vi "Modelo planta H2_V2.vi"() -> ()   [LabVIEW 2024] (continued)
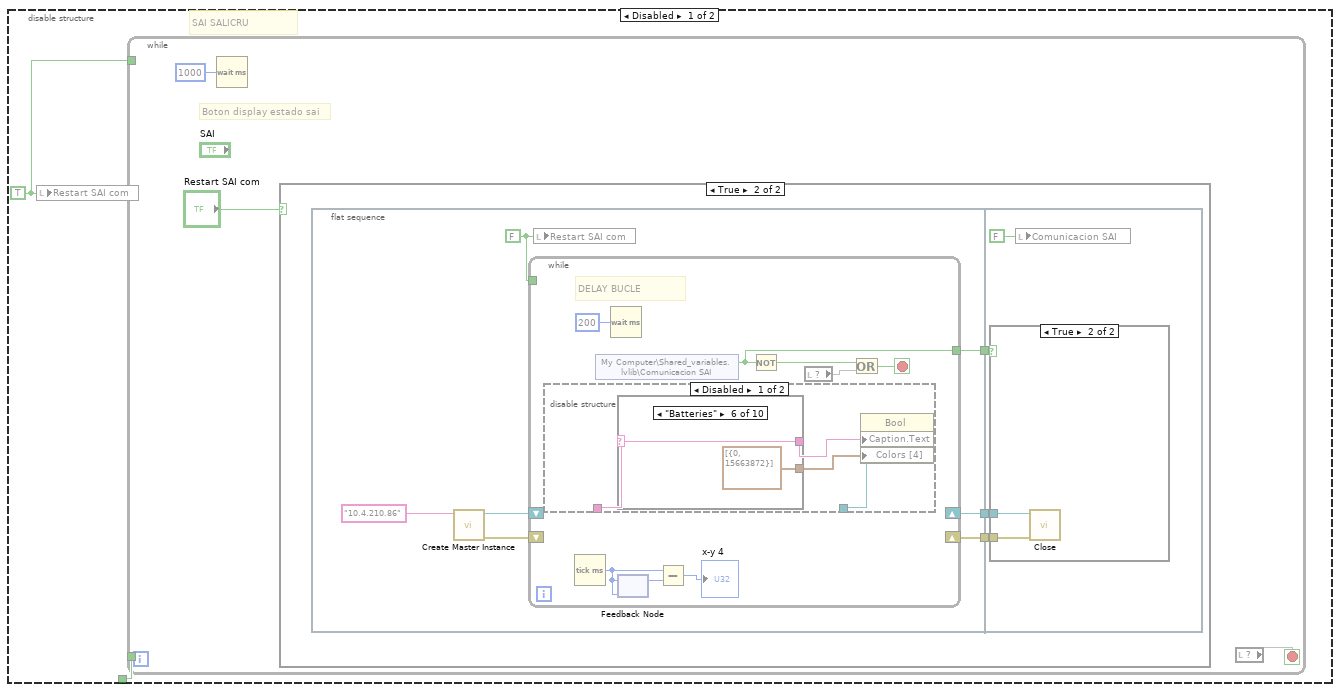
[diagram p2: hidden frame]
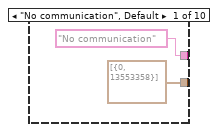
[diagram p4: hidden frame]
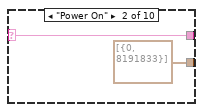
[diagram p5: hidden frame]
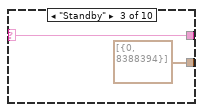
[diagram p6: hidden frame]
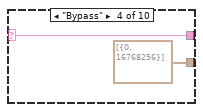
[diagram p7: hidden frame]
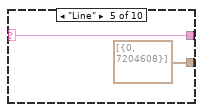
[diagram p8: hidden frame]
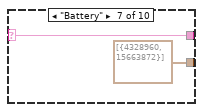
[diagram p9: hidden frame]
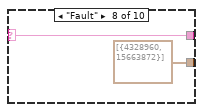
[diagram p10: hidden frame]
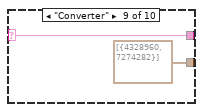
[diagram p11: hidden frame]
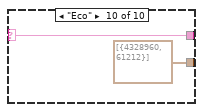
[diagram p12: hidden frame]
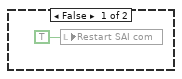
[diagram p14: hidden frame]
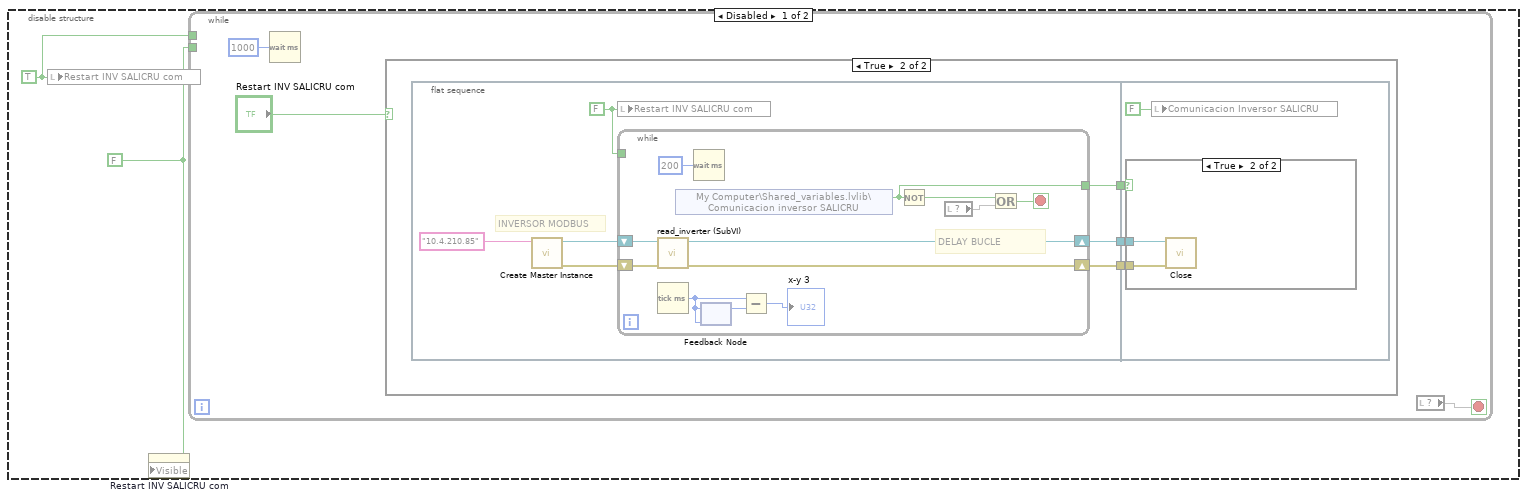
[diagram p15: hidden frame]
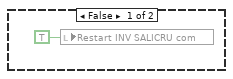
[diagram p17: hidden frame]
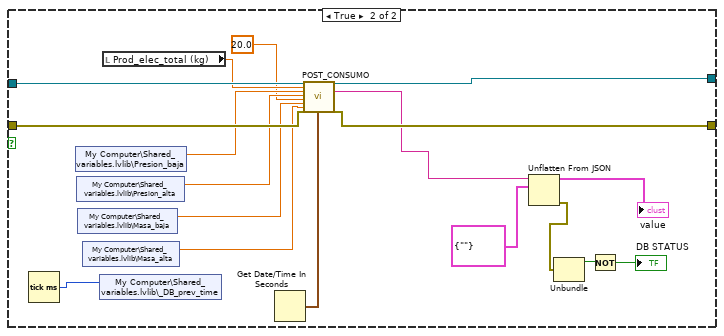
[diagram p18: hidden frame]
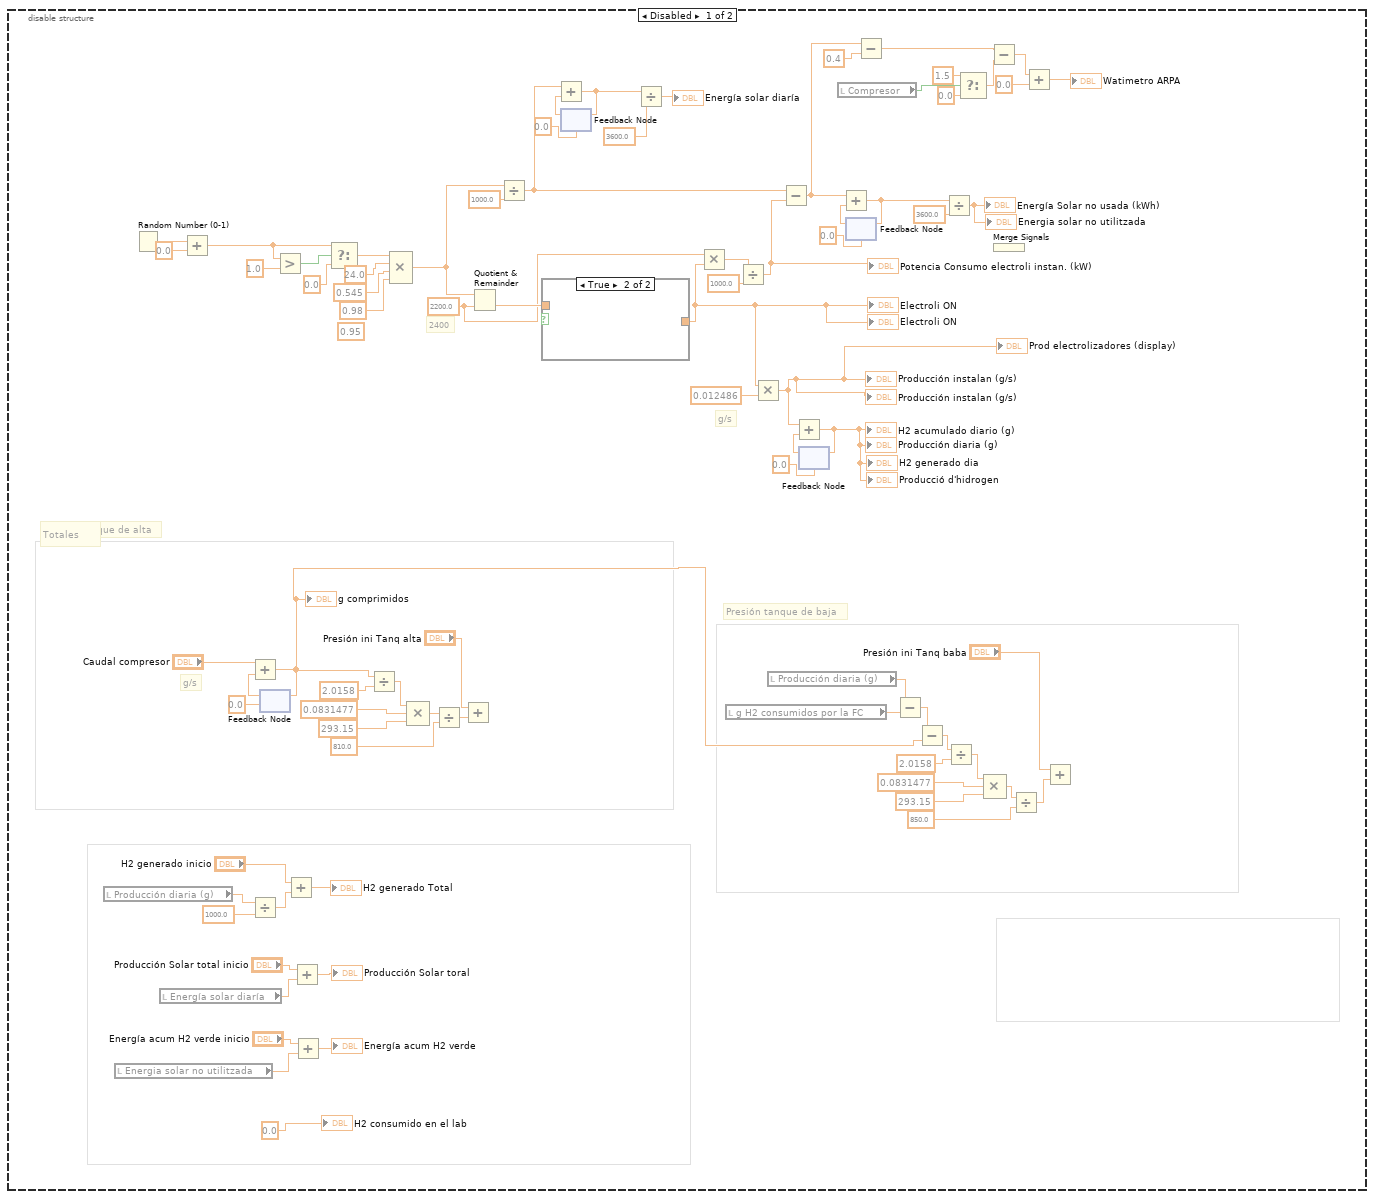
[diagram p20: hidden frame]
                    disable-tunnel: _ -> [w170 _]
                    disable-tunnel: _ -> [w167 _]
                    frame Disabled {
                      n87 = case shown="\"Batteries\"" w170 {
                        selector: w170 -> [_ w174 w176 w178 w180 w182 w184 w186 w188 w190]
                        tunnel: ["No communication" w174 w176 w178 w180 w182 w184 w186 w188 w190] -> w169
                        tunnel: [cluster{u32, u32}[] [{0, 13553358}] ("Colors [4]") cluster{u32, u32}[] [{0, 8191833}] ("Colors [4]") cluster{u32, u32}[] [{0, 8388394}] ("Colors [4]") cluster{u32, u32}[] [{0, 16768256}] ("Colors [4]") cluster{u32, u32}[] [{0, 7204608}] ("Colors [4]") cluster{u32, u32}[] [{0, 15663872}] ("Colors [4]") cluster{u32, u32}[] [{4328960, 15663872}] ("Colors [4]") cluster{u32, u32}[] [{4328960, 15663872}] ("Colors [4]") cluster{u32, u32}[] [{4328960, 7274282}] ("Colors [4]") cluster{u32, u32}[] [{4328960, 61212}] ("Colors [4]")] -> w168
                        frame "No communication", Default {
                        }
                        frame "Power On" {
                        }
                        frame "Standby" {
                        }
                        frame "Bypass" {
                        }
                        frame "Line" {
                        }
                        frame "Batteries" {
                        }
                        frame "Battery" {
                        }
                        frame "Fault" {
                        }
                        frame "Converter" {
                        }
                        frame "Eco" {
                        }
                      }
                      n88 = property class="Bool"(reference=w167, "Caption.Text"=w169, "Colors [4]"=w168) -> ()  [unwired: 1 in, 2 out]
                    }
                    frame Enabled {
                    }
                  }
                  n89 = Tick Count (ms)() -> (millisecond timer value=w164:u32)
                  n90 = shared-variable "My Computer\\Shared_variables.lvlib\\Comunicacion SAI"() -> (w160:bool)  [unwired: 1 in, 1 out]
                  n91 = Wait (ms)(milliseconds to wait=u32 200) -> ()  [unwired: 1 out]
                  n92 = feedback #6(w164) -> (w163:u32)
                  n93 = feedback-in #6(w164) -> ()
                  n94 = Subtract(x=w164, y=w163) -> (x-y=→"x-y 4":u32)
                  n95 = Not(x=w160) -> (.not. x?=w161:bool)
                  n96 = local read item#-1() -> (w159)
                  n97 = Or(x=w161, y=w159) -> (x .or. y?=w165:bool)
                }
                n98 = local write "Restart SAI com"(w153) -> ()
              }
              frame #1 {
                n99 = case shown="True" w191 {
                  tunnel: w194 -> [_ w197]
                  tunnel: w193 -> [_ w196]
                  frame False {
                    n100 = local write "Restart SAI com"(TRUE ("Restart SAI com")) -> ()
                  }
                  frame True {
                    n101 = call-dynamic "Close.vi"("error in (no error)"=w197, "Modbus master in"=w196) -> ()  [unwired: 9 in, 1 out]
                  }
                }
                n102 = local write "Comunicacion SAI"(FALSE) -> ()
              }
            }
          }
        }
        n103 = local read item#-1() -> (w146)
      }
    }
    frame Enabled {
    }
  }
  n104 = flat-sequence {
    tunnel: [w245] -> w26
    tunnel: [w240] -> w25
    tunnel: [w239] -> w24
    tunnel: [w220] -> w23
    tunnel: [map{string, dbl}[] []] -> w22
    tunnel: [w217] -> w21
    tunnel: [w216] -> w20
    tunnel: [w214] -> w19
    tunnel: [w213] -> w18
    tunnel: [w211] -> w17
    tunnel: [w210] -> w16
    tunnel: [w202] -> w15
    tunnel: [w201] -> w4
    tunnel: [w200] -> w3
    tunnel: w26 -> [_]
    tunnel: w25 -> [w269]
    tunnel: w24 -> [w270]
    tunnel: w23 -> [w252]
    tunnel: w22 -> [_]
    tunnel: w21 -> [w254]
    tunnel: w20 -> [w253]
    tunnel: w19 -> [w260]
    tunnel: w18 -> [w259]
    tunnel: w17 -> [w264]
    tunnel: w16 -> [w263]
    tunnel: w15 -> [w273]
    tunnel: [w268] -> w14
    tunnel: [w267] -> w13
    tunnel: [w266] -> w12
    tunnel: [w265] -> w11
    tunnel: [w261] -> w10
    tunnel: [w262] -> w9
    tunnel: [w258] -> w8
    tunnel: [w257] -> w7
    tunnel: [w256] -> w6
    tunnel: [w255] -> w5
    tunnel: w4 -> [w249]
    tunnel: w3 -> [w248]
    tunnel: [w247] -> w2
    tunnel: [w246] -> w1
    tunnel: w14 -> [w413]
    tunnel: w13 -> [w412]
    tunnel: w12 -> [w411]
    tunnel: w11 -> [w410]
    tunnel: w10 -> [w409]
    tunnel: w9 -> [w408]
    tunnel: w8 -> [w407]
    tunnel: w7 -> [w406]
    tunnel: w6 -> [w405]
    tunnel: w5 -> [w404]
    tunnel: w2 -> [w402]
    tunnel: w1 -> [w401]
    frame #0 {
      w244 = dynamicdata[] [] ("History Data")
      w245 = dbl[] [] ("History Data")
      # "INICIALIZACIÓN"
      n105 = property on="Restart SAI com" class="Bool (strict)"("Visible"=FALSE) -> ()  [unwired: 2 in, 2 out]
      n106 = Get Date/Time In Seconds() -> (seconds since 1Jan1904=w208:timestamp)
      n107 = control-ref of="E2.1"() -> (w230:refnum<vi>)
      n108 = control-ref of="E2.1.2"() -> (w231:refnum<vi>)
      n109 = control-ref of="E2.2"() -> (w233:refnum<vi>)
      n110 = control-ref of="E2.2.2"() -> (w234:refnum<vi>)
      n111 = control-ref of="E2.3.2"() -> (w236:refnum<vi>)
      n112 = control-ref of="E2.3"() -> (w237:refnum<vi>)
      n113 = control-ref of="E1.1,2"() -> (w226:refnum<vi>)
      n114 = control-ref of="E1.1"() -> (w225:refnum<vi>)
      n115 = control-ref of="E1.2"() -> (w223:refnum<vi>)
      n116 = control-ref of="E1.2.2"() -> (w222:refnum<vi>)
      n117 = control-ref of="E1.3.2"() -> (w227:refnum<vi>)
      n118 = control-ref of="E1.3"() -> (w228:refnum<vi>)
      n119 = Format Date/Time String(time format string (%c)="%Y_%m_%d_%H_%M", seconds (now)=w208) -> (date/time string=w206:string)  [unwired: 1 in]
      n120 = Build Array(w230, w231) -> (w232:refnum<vi>[])
      n121 = Build Array(w233, w234) -> (w235:refnum<vi>[])
      n122 = Build Array(w236, w237) -> (w238:refnum<vi>[])
      n123 = Build Array(w226, w225) -> (w224:refnum<vi>[])
      n124 = Build Array(w223, w222) -> (w221:refnum<vi>[])
      n125 = Build Array(w227, w228) -> (w229:refnum<vi>[])
      n126 = Build Array(w224, w221, w229, w232, w235, w238) -> (w220:refnum<vi>[][])
      n127 = Concatenate Strings("C:\\Users\\h2.lab\\Documents\\LabVIEW My DATA\\" ("string"), w206, "_data Planta Pilot.tdms" ("string")) -> (w207:string)
      n128 = call-poly <vilib>:"Create Master Instance.vi"("address"="10.4.210.79") -> ("error out"=w216:errorcluster, "TCP master instance"=w217:refnum<class "Modbus Master.lvclass">)  [unwired: 9 in]
      n129 = call-poly <vilib>:"Create Master Instance.vi"("address"="10.4.210.85") -> ("error out"=w213:errorcluster, "TCP master instance"=w214:refnum<class "Modbus Master.lvclass">)  [unwired: 9 in]
      n130 = call-poly <vilib>:"Create Master Instance.vi"("address"="10.4.210.86") -> ("error out"=w210:errorcluster, "TCP master instance"=w211:refnum<class "Modbus Master.lvclass">)  [unwired: 9 in]
      n131 = String To Path(string=w207) -> (path=w202:path)
      n132 = call <vilib>:"Connect.vi"("trust any server (F)"=TRUE, "security policy"=T2 {"message mode"=enum."None", "security"=enum."Basic256"}, "server endpoint URL"="opc.tcp://10.4.210.54:4841") -> ("error out"=w240:errorcluster, "OPC UA client refnum out"=w239:T7)  [unwired: 6 in, 1 out]
      n133 = property on="Potencia Solar Instanta (kW)" class="WFChart (strict)"("History Data"=w245) -> ()  [unwired: 2 in, 2 out]
      n134 = property on="Potencia Consumo electroli instan. (kW)" class="WFChart (strict)"("History Data"=w245) -> ()  [unwired: 2 in, 2 out]
      n135 = property on="Electroli ON" class="WFChart (strict)"("History Data"=w245) -> ()  [unwired: 2 in, 2 out]
      n136 = property on="Producción instalan (g/s)" class="WFChart (strict)"("History Data"=w245) -> ()  [unwired: 2 in, 2 out]
      n137 = property on="H2 acumulado diario (g)" class="WFChart (strict)"("History Data"=w245) -> ()  [unwired: 2 in, 2 out]
      n138 = property on="Energía Solar no usada (kWh)" class="WFChart (strict)"("History Data"=w245) -> ()  [unwired: 2 in, 2 out]
      n139 = property on="P tanq baja (barg)" class="WFChart (strict)"("History Data"=w245) -> ()  [unwired: 2 in, 2 out]
      n140 = property on="Producció d'hidrogen" class="WFChart (strict)"("History Data"=w245) -> ()  [unwired: 2 in, 2 out]
      n141 = property on="Energia solar no utilitzada" class="WFChart (strict)"("History Data"=w245) -> ()  [unwired: 2 in, 2 out]
      n142 = property on="Potència inversor solar" class="WFChart (strict)"("History Data"=w244) -> ()  [unwired: 2 in, 2 out]
      n143 = property on="Pressió tanc baixa" class="WFChart (strict)"("History Data"=w244) -> ()  [unwired: 2 in, 2 out]
      n144 = call "Init.vi"("Port"=u32 8000, "IP"="10.4.210.42") -> ("error out"=w200:errorcluster, "DB_API.lvclass 2"=w201:refnum<class "DB_API.lvclass">)  [unwired: 8 in]
    }
    frame #1 {
      # "PLC"
      # "ELECTROLIZADORES"
      # "ALMACENAMIENTO DE DATOS"
      n145 = node-c288() -> (w275:T3)  [unwired: 4 in]
      n146 = timed-loop {
        timing: w275 -> [_]
        timing-out: [_] -> w274
        stop <- w343 stop-if-true
        # "VISUALIZACIÓN"
        n147 = node-c288() -> ()  [unwired: 1 in, 1 out]
        n148 = shared-variable "My Computer\\Shared_variables.lvlib\\Baliza_amarilla"() -> (→"Baliza amarilla":bool)  [unwired: 1 in, 1 out]
        n149 = shared-variable "My Computer\\Shared_variables.lvlib\\Baliza_roja"() -> (→"Baliza roja":bool)  [unwired: 1 in, 1 out]
        n150 = shared-variable "My Computer\\Shared_variables.lvlib\\ELYs_Produccio_Total"() -> (w337:dbl[])  [unwired: 1 in, 1 out]
        "ELYs_Produccio_1" <- w337
        n151 = shared-variable "My Computer\\Shared_variables.lvlib\\Baliza_verde"() -> (→"Baliza verde":bool)  [unwired: 1 in, 1 out]
        n152 = shared-variable "My Computer\\Shared_variables.lvlib\\Compresor"() -> (→"Compresor":bool)  [unwired: 1 in, 1 out]
        n153 = shared-variable "My Computer\\Shared_variables.lvlib\\EV3"() -> (→"EV3":bool)  [unwired: 1 in, 1 out]
        n154 = shared-variable "My Computer\\Shared_variables.lvlib\\EV1"() -> (→"EV1":bool)  [unwired: 1 in, 1 out]
        n155 = shared-variable "My Computer\\Shared_variables.lvlib\\ELYs_Produccio_inst"() -> (w341:dbl[])  [unwired: 1 in, 1 out]
        "ELYs_Produccio_2" <- w341
        n156 = shared-variable "My Computer\\Shared_variables.lvlib\\EV2"() -> (→"EV2":bool)  [unwired: 1 in, 1 out]
        n157 = shared-variable "My Computer\\Shared_variables.lvlib\\Comunicacion SAI"() -> (→"Comunicacion SAI":bool)  [unwired: 1 in, 1 out]
        n158 = local read "stop"() -> (w342:bool)
        n159 = shared-variable "My Computer\\Shared_variables.lvlib\\Stop"(w342) -> ()  [unwired: 1 in, 1 out]
        n160 = shared-variable "My Computer\\Shared_variables.lvlib\\EV5"() -> (→"EV5":bool)  [unwired: 1 in, 1 out]
        n161 = shared-variable "My Computer\\Shared_variables.lvlib\\EV4"() -> (→"EV4":bool)  [unwired: 1 in, 1 out]
        n162 = shared-variable "My Computer\\Shared_variables.lvlib\\EV6"() -> (→"EV6":bool)  [unwired: 1 in, 1 out]
        n163 = shared-variable "My Computer\\Shared_variables.lvlib\\Termic_extractors"() -> (→"Tèrmic\nExtractors":bool)  [unwired: 1 in, 1 out]
        n164 = shared-variable "My Computer\\Shared_variables.lvlib\\rele_seguretat"() -> (→"Relé Seguretat":bool)  [unwired: 1 in, 1 out]
        n165 = shared-variable "My Computer\\Shared_variables.lvlib\\Sobretensions"() -> (→"Sobretensions":bool)  [unwired: 1 in, 1 out]
        n166 = for {
          tunnel: w337 -> [w385] mode=indexing
          shift-right: [w389] -> w334
          shift-left: 0.0 -> [w390]
          w386 = 0.0 ("x")
          n167 = Greater Or Equal?(x=w385, y=w386) -> (x >= y?=w387:bool)
          n168 = Select(t=w385, s=w387, f=w386) -> (s? t:f=w388:dbl)
          n169 = Add(x=w388, y=w390) -> (x+y=w389:dbl)
        }
        n170 = shared-variable "My Computer\\Shared_variables.lvlib\\Comunicacion inversor SALICRU"() -> (→"Comunicacion Inversor SALICRU":bool)  [unwired: 1 in, 1 out]
        n171 = for {
          tunnel: w341 -> [w391] mode=indexing
          shift-right: [w395] -> w339
          shift-left: 0.0 -> [w396]
          w392 = 0.0 ("x")
          n172 = Greater Or Equal?(x=w391, y=w392) -> (x >= y?=w393:bool)
          n173 = Select(t=w391, s=w393, f=w392) -> (s? t:f=w394:dbl)
          n174 = Add(x=w394, y=w396) -> (x+y=w395:dbl)
        }
        "Prod_elec_inst (g/s)" <- w339
        n175 = shared-variable "My Computer\\Shared_variables.lvlib\\Masa_alta"() -> (→"masa total G Kg" →"masa total G Kg 2":dbl)  [unwired: 1 in, 1 out]
        n176 = shared-variable "My Computer\\Shared_variables.lvlib\\Presion_alta"() -> (→"P tanq alta (barg)" →"P alta" →"P alta 2":dbl)  [unwired: 1 in, 1 out]
        n177 = Multiply(x=w334, y=0.0899) -> (x*y=w333:dbl)
        n178 = Divide(x=w333, y=1000.0) -> (x/y=→"Prod_elec_total (kg)":dbl)
        n179 = shared-variable "My Computer\\Shared_variables.lvlib\\Presion_baja"() -> (w358:dbl)  [unwired: 1 in, 1 out]
        "P tanq baja (barg)" <- w358
        "P baja" <- w358
        "P baja 2" <- w358
        n180 = shared-variable "My Computer\\Shared_variables.lvlib\\Potencia solar"() -> (w363:dbl)  [unwired: 1 in, 1 out]
        "Potencia Solar Instanta (kW)" <- w363
        "Potenica Solar (Display)" <- w363
        "Potenica Solar (Display) 2" <- w363
        n181 = shared-variable "My Computer\\Shared_variables.lvlib\\Masa_baja"() -> (→"masa total P Kg" →"masa total P Kg  2":dbl)  [unwired: 1 in, 1 out]
        n182 = shared-variable "My Computer\\Shared_variables.lvlib\\FC_Consumo_g"() -> (→"g H2 consumidos por la FC":dbl)  [unwired: 1 in, 1 out]
        n183 = shared-variable "My Computer\\Shared_variables.lvlib\\Potencia SAI"() -> (→"Potenica SAI (Display) 3":dbl)  [unwired: 1 in, 1 out]
        n184 = shared-variable "My Computer\\Shared_variables.lvlib\\FC_Produccion"() -> (→"Producción FC":dbl)  [unwired: 1 in, 1 out]
        n185 = shared-variable "My Computer\\Shared_variables.lvlib\\Temperatura"() -> (→"Temperatura":dbl)  [unwired: 1 in, 1 out]
        n186 = shared-variable "My Computer\\Shared_variables.lvlib\\Salida Vs"() -> (→"Salida Vs":dbl)  [unwired: 1 in, 1 out]
        n187 = shared-variable "My Computer\\Shared_variables.lvlib\\Salida Vt"() -> (→"Salida Vt":dbl)  [unwired: 1 in, 1 out]
        n188 = shared-variable "My Computer\\Shared_variables.lvlib\\Salida Vr"() -> (→"Salida Vr":dbl)  [unwired: 1 in, 1 out]
        n189 = shared-variable "My Computer\\Shared_variables.lvlib\\Corriente T"() -> (→"Corriente T":dbl)  [unwired: 1 in, 1 out]
        n190 = shared-variable "My Computer\\Shared_variables.lvlib\\Corriente R"() -> (→"Corriente R":dbl)  [unwired: 1 in, 1 out]
        n191 = shared-variable "My Computer\\Shared_variables.lvlib\\Corriente S"() -> (→"Corriente S":dbl)  [unwired: 1 in, 1 out]
        n192 = shared-variable "My Computer\\Shared_variables.lvlib\\Humedad"() -> (→"Humedad":dbl)  [unwired: 1 in, 1 out]
        n193 = Merge Signals(w363) -> (→"Potència inversor solar":dynamicdata)
        n194 = Merge Signals(w358) -> (→"Pressió tanc baixa":dynamicdata)
        n195 = shared-variable "My Computer\\Shared_variables.lvlib\\CO2"() -> (→"CO2":dbl)  [unwired: 1 in, 1 out]
        n196 = shared-variable "My Computer\\Shared_variables.lvlib\\H2S"() -> (→"H2S":dbl)  [unwired: 1 in, 1 out]
        n197 = shared-variable "My Computer\\Shared_variables.lvlib\\TVOC"() -> (→"TVOC":dbl)  [unwired: 1 in, 1 out]
        n198 = shared-variable "My Computer\\Shared_variables.lvlib\\NO2"() -> (→"NO2":dbl)  [unwired: 1 in, 1 out]
        n199 = shared-variable "My Computer\\Shared_variables.lvlib\\SO2"() -> (→"SO2":dbl)  [unwired: 1 in, 1 out]
        n200 = shared-variable "My Computer\\Shared_variables.lvlib\\CO"() -> (→"CO":dbl)  [unwired: 1 in, 1 out]
        n201 = shared-variable "My Computer\\Shared_variables.lvlib\\O2"() -> (→"O2":dbl)  [unwired: 1 in, 1 out]
        n202 = shared-variable "My Computer\\Shared_variables.lvlib\\O3"() -> (→"O3":dbl)  [unwired: 1 in, 1 out]
        n203 = local read "stop"() -> (w343:bool)
        n204 = node-c288() -> ()  [unwired: 1 in, 1 out]
      }
      n205 = node-c288() -> (w251:T3)  [unwired: 4 in]
      n206 = timed-loop {
        timing: w251 -> [_]
        timing-out: [_] -> w250
        shift-right: [w282] -> w247
        shift-left: w249 -> [w284]
        shift-right: [w281] -> w246
        shift-left: w248 -> [w283]
        stop <- w285 stop-if-true
        n207 = node-c288() -> ()  [unwired: 1 in, 1 out]
        n208 = shared-variable "My Computer\\Shared_variables.lvlib\\_DB_prev_time"() -> (w279:i32)  [unwired: 1 in, 1 out]
        n209 = Tick Count (ms)() -> (millisecond timer value=w280:u32)
        n210 = Subtract(x=w280, y=w279) -> (x-y=w278:u32)
        n211 = Greater Or Equal?(x=w278, y=u32 600000) -> (x >= y?=w276:bool)
        n212 = case shown="False" w276 {
          tunnel: w284 -> [w286 w305]
          tunnel: w283 -> [w287 w304]
          tunnel: [w286 w303] -> w282
          tunnel: [w287 w295] -> w281
          frame False {
          }
          frame True {
            n213 = Tick Count (ms)() -> (millisecond timer value=w288:u32)
            n214 = shared-variable "My Computer\\Shared_variables.lvlib\\Presion_baja"() -> (w300:dbl)  [unwired: 1 in, 1 out]
            n215 = shared-variable "My Computer\\Shared_variables.lvlib\\Presion_alta"() -> (w299:dbl)  [unwired: 1 in, 1 out]
            n216 = shared-variable "My Computer\\Shared_variables.lvlib\\Masa_baja"() -> (w297:dbl)  [unwired: 1 in, 1 out]
            n217 = shared-variable "My Computer\\Shared_variables.lvlib\\Masa_alta"() -> (w296:dbl)  [unwired: 1 in, 1 out]
            n218 = shared-variable "My Computer\\Shared_variables.lvlib\\_DB_prev_time"(w288) -> ()  [unwired: 1 in, 1 out]
            n219 = local read "Prod_elec_total (kg)"() -> (w301:dbl)
            n220 = Get Date/Time In Seconds() -> (seconds since 1Jan1904=w302:timestamp)
            n221 = call "POST_CONSUMO.vi"("DB_API.lvclass"=w305, "Produccion total"=w301, "Presion baja"=w300, "Presion alta"=w299, "Temperatura"=20.0, "Masa baja"=w297, "Masa alta"=w296, "error in (no error)"=w304, "Time Stamp"=w302) -> ("DB_API.lvclass 2"=w303:refnum<class "DB_API.lvclass">, "body"=w291:string, "error out"=w295:errorcluster)  [unwired: 16 in]
            n222 = Unflatten From JSON(JSON string=w291, type and defaults=cluster{"message":string} {"message"=""}) -> (value=→"value":cluster{"message":string}, error out=w290:errorcluster)  [unwired: 5 in]
            n223 = Unbundle(w290) -> ("status"=w289:bool)  [unwired: 2 out]
            n224 = Not(x=w289) -> (.not. x?=→"DB STATUS":bool)
          }
        }
        n225 = shared-variable "My Computer\\Shared_variables.lvlib\\Stop"() -> (w285:bool)  [unwired: 1 in, 1 out]
        n226 = node-c288() -> ()  [unwired: 1 in, 1 out]
      }
      n227 = while {
        tunnel: w273 -> [w311]
        stop <- "stop" stop-if-true
        n228 = call "Elapsed Time"("Auto Reset"=TRUE) -> ("Time has Elapsed"=w313:bool)  [unwired: 11 in, 7 out]
        n229 = Wait (ms)(milliseconds to wait=u32 500) -> ()  [unwired: 1 out]
        n230 = case shown="True" w313 {
          tunnel: w311 -> [_ w323]
          frame False {
          }
          frame True {
            w330 = "Energia" ("group name in (Untitled)")
            n231 = local read "Potenica Solar (Display) 2"() -> (w328:dbl)
            n232 = local read "Potenica SAI (Display) 3"() -> (w320:dbl)
            n233 = Build Array(w328, w320) -> (w317:dbl[])
            n234 = TDMS Open(10:T6."open or create" ("operation (0:open)"), 11:w323) -> (0:w326:errorcluster, 3:w327:refnum<k34>)  [unwired: 5 in]
            n235 = call "Save_PLC (SubVI).vi"("error in (no error)"=w326, "Refnum in"=w327) -> ("error out"=w325:errorcluster, "Refnum out"=w324:refnum<k34>)  [unwired: 8 in]
            n236 = Build Array(w317) -> (w316:dbl[][])
            n237 = call "Save_Time (SubVI).vi"("error in (no error)"=w325, "group name in (Untitled)"=w330, "Refnum in"=w324) -> ("error out"=w321:errorcluster, "Refnum out"=w322:refnum<k34>)  [unwired: 7 in]
            n238 = Transpose 2D Array(2D array=w316) -> (transposed array=w315:dbl[][])
            n239 = TDMS Write(0:w322, 5:w330, 7:string[] ["Potencia Solar (kW)", "Potencia SAI (%)", "Prod. ElY (g/s)"] ("channel name(s) in (Untitled)"), 9:w315, 11:w321) -> (4:w319:refnum<k34>, 15:w318:errorcluster)  [unwired: 1 in, 2 out]
            n240 = TDMS Close(8:w318, 11:w319) -> ()  [unwired: 2 out]
          }
        }
      }
      n241 = control-ref of="SAI"() -> (w271:refnum<vi>)
      n242 = call "(SubVI)SAI_PANEL_CODIGO.vi"("Modbus Master in"=w264, "SAI"=w271, "error in (no error)"=w263) -> ("Modbus Master out"=w261:refnum<class "Modbus Master.lvclass">, "error out"=w262:errorcluster)  [unwired: 10 in, 5 out]
      n243 = call "Reading_ELYs_OPC_UA (SubVI).vi"("Array 4"=w252, "error in (no error)"=w269, "Refnum in"=w270) -> ("error out"=w266:errorcluster, "Refnum out"=w267:T7)  [unwired: 7 in]
      n244 = call "read_inverter (SubVI).vi"("error in (no error)"=w259, "Modbus Master in"=w260) -> ("error out"=w257:errorcluster, "Modbus Master out"=w258:refnum<class "Modbus Master.lvclass">)  [unwired: 8 in]
      n245 = call "read_s7_1200 (SubVI).vi"("error in (no error)"=w269, "Refnum in"=w270) -> ("error out"=w265:errorcluster, "Refnum out"=w268:T7)  [unwired: 8 in]
      n246 = call "Aire (subVI).vi"("milliseconds to wait"=u32 4000, "error in (no error)"=w253, "Modbus Master in"=w254) -> ("error out"=w255:errorcluster, "Modbus Master out"=w256:refnum<class "Modbus Master.lvclass">)  [unwired: 6 in, 1 out]
      n247 = node-c288(w274) -> ()  [unwired: 1 out]
      n248 = node-c288(w250) -> ()  [unwired: 1 out]
    }
    frame #2 {
      # "FINAL"
      n249 = call <vilib>:"Disconnect.vi"("error in (no error)"=w410, "OPC UA client refnum in"=w413) -> ()  [unwired: 9 in, 1 out]
      n250 = call <vilib>:"Disconnect.vi"("error in (no error)"=w411, "OPC UA client refnum in"=w412) -> ()  [unwired: 9 in, 1 out]
      n251 = call-dynamic "Close.vi"("error in (no error)"=w406, "Modbus master in"=w407) -> ()  [unwired: 9 in, 1 out]
      n252 = call-dynamic "Close.vi"("error in (no error)"=w408, "Modbus master in"=w409) -> ()  [unwired: 9 in, 1 out]
      n253 = call-dynamic "Close.vi"("error in (no error)"=w404, "Modbus master in"=w405) -> ()  [unwired: 9 in, 1 out]
      n254 = call "Close.vi"("error in (no error)"=w401, "DB_API.lvclass 2"=w402) -> ()  [unwired: 9 in, 1 out]
      n255 = local write "stop"(FALSE ("stop")) -> ()
    }
  }
